vi "Minhee Analysis.vi"(5 "Data type":T4 items=["AXON", "HEKA", "TEXT"], 7 "Path of File":path=path "C:/Users/KimYG/Desktop/test4.abf") -> ()   [LabVIEW 2017]
uses:
  Data type_new.ctl
  <vilib>/Utility/config.llb/Config Data RefNum.ctl
  Polarity.ctl
  <vilib>/Utility/sysdir.llb/System Directory Type.ctl
  Minhee analysis parameter_new.ctl
  <vilib>/Utility/miscctls.llb/LVRowAndColumnTypeDef.ctl
  <vilib>/Analysis/3filter.llb/Savitzky-Golay Filter (DBL).vi
  <vilib>/addons/Wavelet Analysis/application.llb/WA Multiscale Peak Detection (Array).vi
  <vilib>/Utility/file.llb/Write Delimited Spreadsheet (DBL).vi
  <vilib>/Analysis/NI_AALBase.lvlib
  <vilib>/addons/_Advanced Signal Processing/NI_AdvSigProcWA.lvlib
  <vilib>/Utility/config.llb/NI_LVConfig.lvlib
  <vilib>/Analysis/NI_AALPro.lvlib
panel:
  out "History log":string
  in  "Offset":bool
  in  "Event Detection Parameter":cluster{"Minimal Amplitude":dbl, "Polarity":T1} {"Polarity" items=["Inward", "Outward"]}
  in  "Screening Parameters":cluster{"Velocity threshold":dbl, " * SD":dbl}
  in  "Redetect":bool
  in  "Derivative":u16(ring) items=["1st", "2nd"]
  in  "Smoothing Parameters":T2={"Polynomial order"=3, "Side points"=35}
  in  "Trace to display":u16(ring) items=["Raw", "Smoothed"]
  out "Averaged Amplitude":dbl[][](graph)
  out "SD of dv/dt":sgl[](graph)
  in  "File Explorer":bool
  in  "Number of Event":i32
  out "StateFileRefnum":T3
  out "End (sec)":string caption="String"
  out "Event":cluster{dbl[], dbl[]}[](graph)
  out "Holding Current":sgl[](graph)
  out "Frequency":string caption="String"
  out "Sweep duration":dbl
  in  "Clipboard":bool
  out "Number of event":i32[][](graph)
  out "Event #":string caption="String"
  out "Begin (sec)":string caption="String"
  out "IEI (sec)":string caption="String"
  out "Amplitude\n     (pA)":string caption="String"
  out "Event #":string caption="String"
  in  "Pin here":bool
  in  "Raw trace":bool
  out "Distribution of amplitude 2":T5(graph) caption="Selected"
  out "Distribution of IEI 2":T5(graph) caption="Selected"
  out "IEI (sec)":string caption="String"
  out "Amplitude\n     (pA)":string caption="String"
  out "CV":sgl[](graph)
  in  "Screening":bool
  out "Derivative of the event":cluster{"X (time)":dbl[], "dX/dt":dbl[]}[](graph)
  in  "Save":bool
  out "Distribution of amplitude":T5(graph) caption="Total"
  out "Distribution of IEI":T5(graph) caption="Total"
  in  "Event #":i16=4 min=0 max=0 step=1
  in  "Delete":bool
  in  "Import":bool
  in  "Sweep #":i32 min=0 max=49 step=1
  out "Event table":string[][](table)
  out "Whole trace":cluster{"Ramp Pattern":dbl[], "X":dbl[]}[](graph)
  # "Result - Total & Selected events"
  # "OFF"
  # "ON"
  # "Total"
  # "Sweep Info."
  # "Event detection parameters"
  # "Action"
  # "Selected"
  # "Smoothing parameters"
  # "Event Table"
  # "Screening parameters"
  # "Explore your data"
  # "Pg Up"
  # "Event"
  # "Pg Dn"
  # "Home"
  # "Sweep"
  # "End"
  # "Number of event to select"
  # "Whole trace"
  # "(pA)"
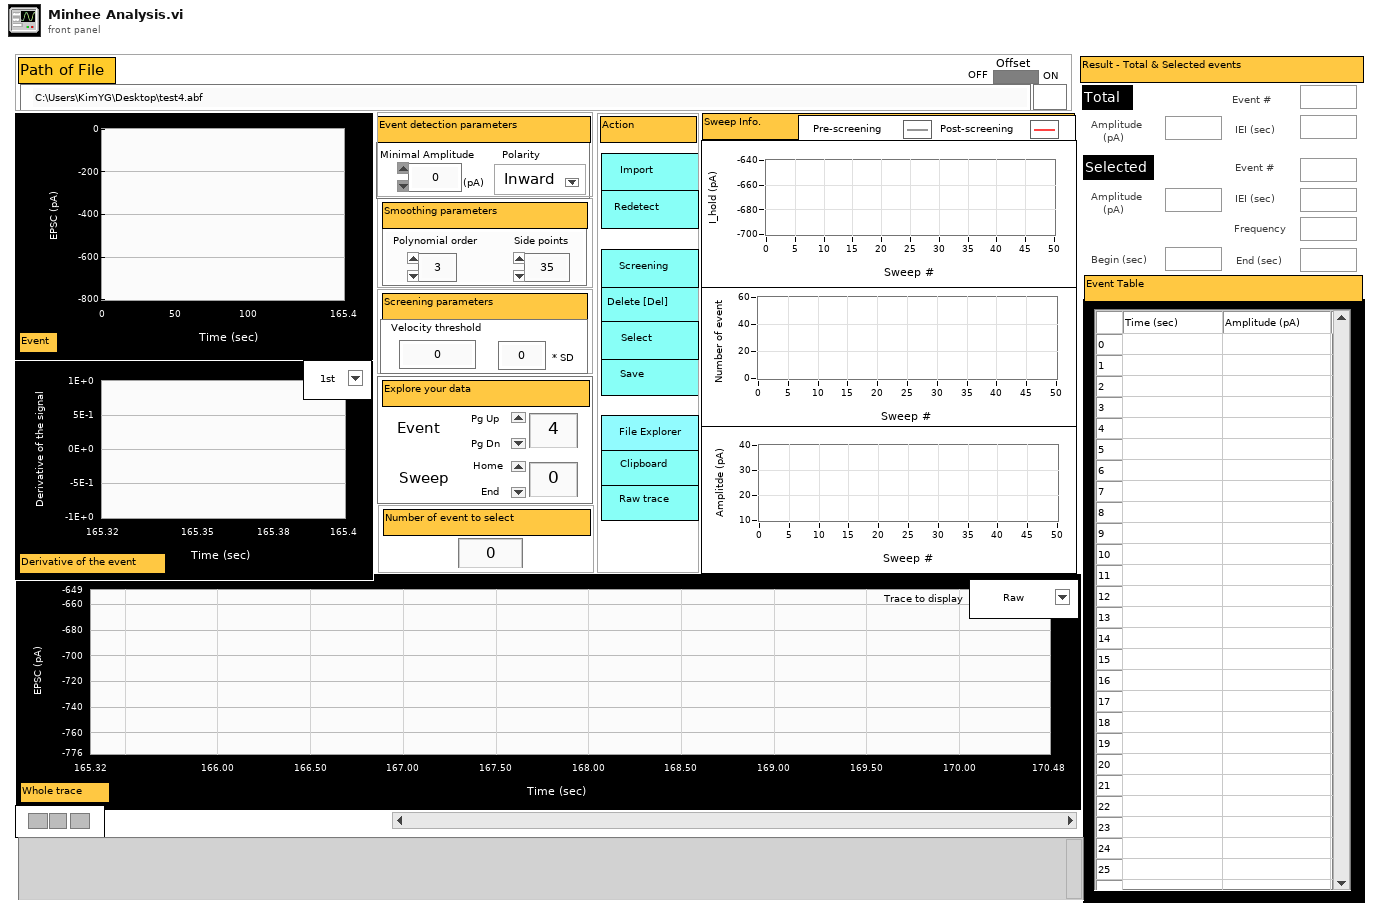
[diagram p1: front panel]
types:
  T1 = typedef "Polarity.ctl" = u16
  T2 = cluster{"Polynomial order":i32, "Side points":i32}
  T3 = typedef "NI_LVConfig.lvlib/Config Data RefNum.ctl" = refnum<k1>
  T4 = typedef "Data type_new.ctl" = u16
  T5 = cluster{"X Values":dbl[], "Histogram: h(x)":i32[]}
  T6 = typedef "Minhee analysis parameter_new.ctl" = cluster{"File Paramters":cluster{"File Path":path, "File Name":string, "Total Length":i32, "Trial Length (ms)":dbl, "Sweep Number":dbl, "Sampling rate":dbl, "Data type":T4}, "Smoothing Parameter":cluster{"Polynomial order":i32, "Side points":i32}, "Event Detection Parameter":cluster{"Event threshold (amplitude)":dbl, "Polarity":T1}, "Screening":cluster{"Screening threshold (dV/dt)":dbl, " * SD":dbl}}
  T7 = cluster{"Total":cluster{"Distribution of IEI":cluster{"X Values":dbl[], "Histogram: h(x)":i32[]}, "Distribution of amplitude":cluster{"X Values":dbl[], "Histogram: h(x)":i32[]}, "Total":cluster{"EVT #":string, "Amplitude":string, "IEI":string}, "Number of event":i32[]}, "Selected":cluster{"Distribution of IEI ":cluster{"X Values":dbl[], "Histogram: h(x)":i32[]}, "Distribution of amplitude":cluster{"X Values":dbl[], "Histogram: h(x)":i32[]}, "Selected":cluster{"EVT #":string, "Amplitude":string, "IEI":string, "Frequency":string}}}
  T8 = cluster{"Distribution of IEI ":cluster{"X Values":dbl[], "Histogram: h(x)":i32[]}, "Distribution of amplitude":cluster{"X Values":dbl[], "Histogram: h(x)":i32[]}, "Selected":cluster{"EVT #":string, "Amplitude":string, "IEI":string, "Frequency":string}}
  T9 = cluster{"detrend? (F)":bool, "threshold frequency":dbl}
  T10 = typedef "System Directory Type.ctl" = i32
  T11 = cluster{"X (time)":dbl[], "I (pA)":dbl[], "dX/dt":dbl[]}
  T12 = typedef "LVRowAndColumnTypeDef.ctl" = cluster{"Row":i32, "Column":i32}
  T13 = cluster{"Sampling rate (Hz)":dbl, "Sweep duration (sec)":dbl, "Unit (A or pA)":u16, "Baseline Offset (pA)":dbl}
  T14 = cluster{"File Path":path, "Cell ID":string, "File Name":string, "Total Length":i32, "Trial Length (ms)":dbl, "Sweep Number":dbl, "Sampling rate":dbl}
  T15 = cluster{"IEI histogram":cluster{"X Values":dbl[], "Histogram: h(x)":i32[]}, "Amplitude histogram":cluster{"X Values":dbl[], "Histogram: h(x)":i32[]}, "Result in Total ":cluster{"Event #":string, "Amplitude ":string, "IEI":string}, i32[]}
  T16 = cluster{"Polynomial order":i32, "Side points":i32}[]
  T17 = cluster{"Histogram Graph":cluster{"X Values":dbl[], "Histogram: h(x)":i32[]}, "Histogram Graph":cluster{"X Values":dbl[], "Histogram: h(x)":i32[]}, cluster{string, "standard deviation":string, "standard deviation":string}, i32[]}
  T18 = cluster{"Histogram Graph":cluster{"X Values":dbl[], "Histogram: h(x)":i32[]}, "Histogram Graph":cluster{"X Values":dbl[], "Histogram: h(x)":i32[]}, cluster{"EVT #":string, "Mean amplitude":string, "Mean IEI":string, "Mean frequency":string}}
  T19 = cluster{"EVT #":string, "Amplitude":string, "IEI":string}
  T20 = cluster{"EVT #":string, "Amplitude":string, "IEI":string, "Frequency":string}
  T21 = cluster{"X (time)":dbl[], "I (pA)":dbl[], "1st derivative":dbl[], "2nd derivative":dbl[]}
  T22 = cluster{"X (time)":dbl[], "2nd derivative":dbl[]}
  T23 = cluster{"X (time)":dbl[], "2nd derivative":dbl[]}[]
  T24 = enum32{"invalid app kind", "Development System", "Run Time System", "Student Edition", "Embedded LabVIEW", "Evaluation", "Custom"}
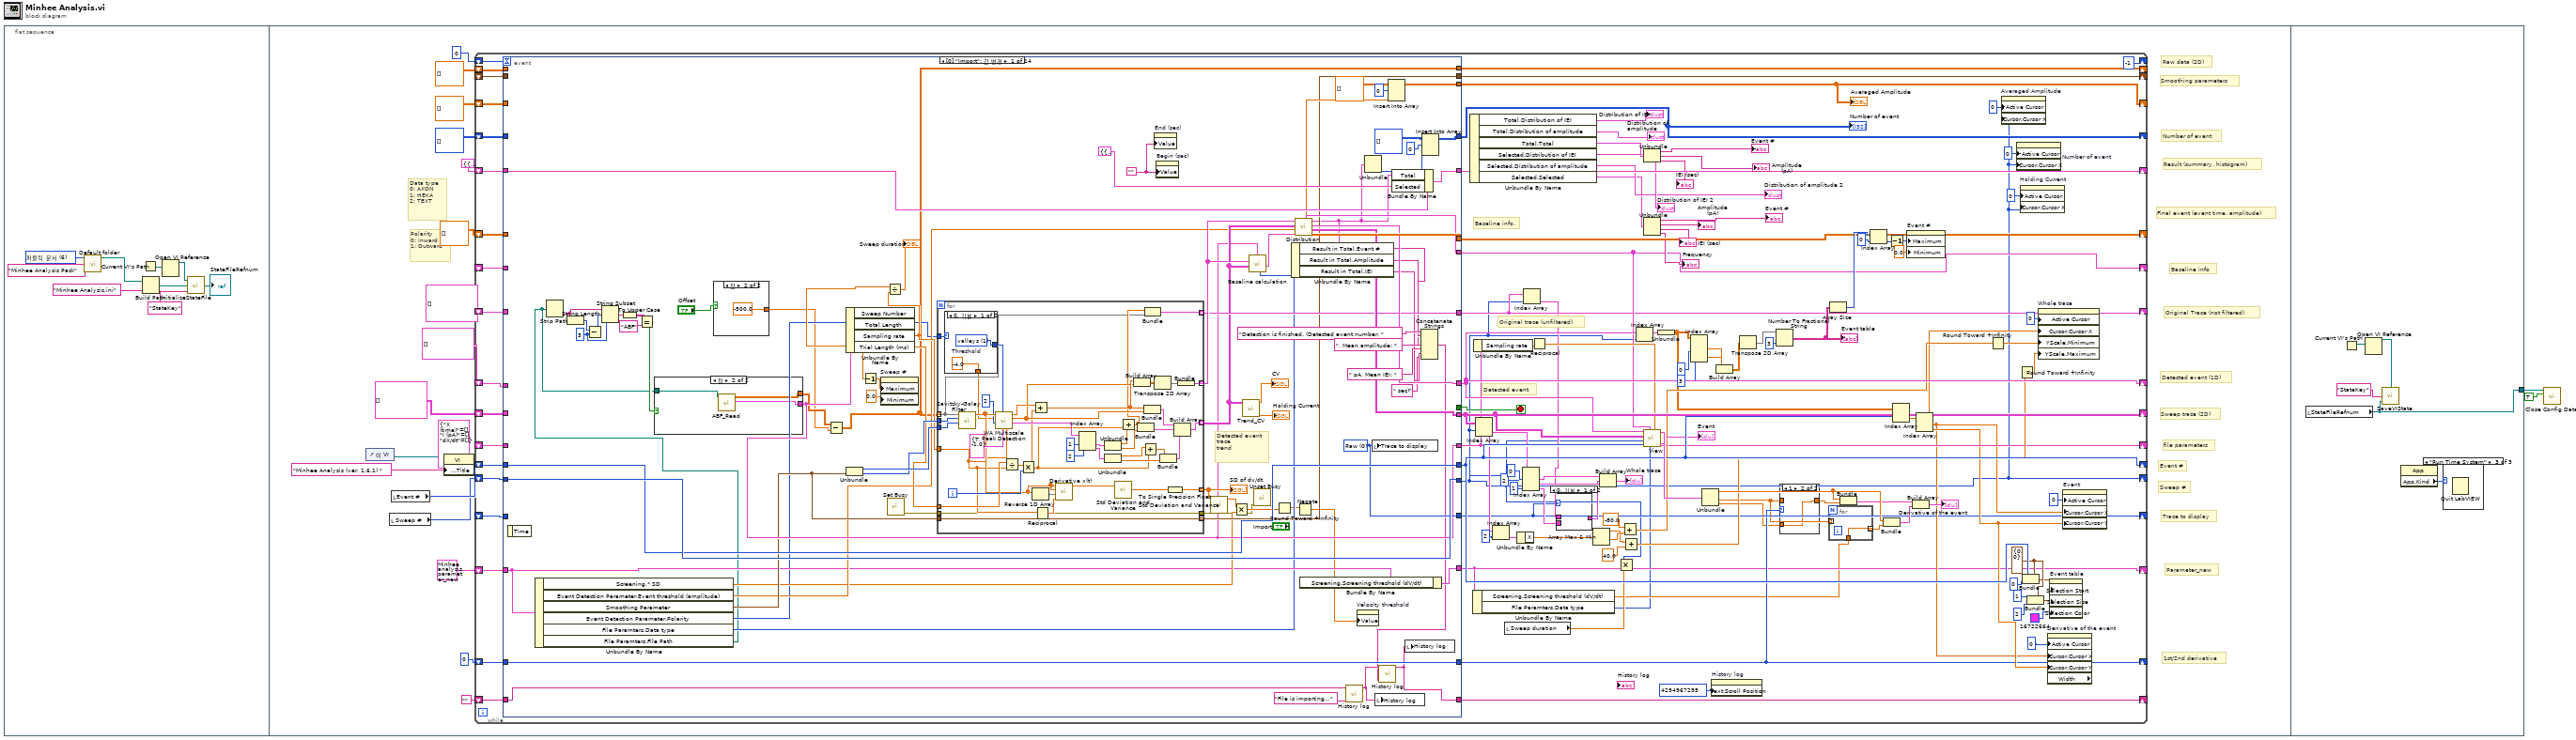
[diagram p0: block diagram]
diagram:
  n1 = flat-sequence {
    tunnel: [w730] -> w1
    frame #0 {
      w9 = T10 6 items=["사용자 홈"=0, "사용자 데스크탑"=1, "사용자 문서"=2, "사용자 어플리케이션 데이터"=3, "사용자 환경"=4, "사용자 임시"=5, "퍼블릭 문서"=6, "퍼블릭 어플리케이션 데이터"=7, "퍼블릭 환경"=8, "퍼블릭 캐시"=13, "시스템 코어 라이브러리"=9, "시스템 설치된 라이브러리"=10, "어플리케이션 파일"=11, "부팅 볼륨 루트"=12] ("system directory type")
      n2 = call <userlib>:"Default folder.vi"("Folder name"="Minhee Analysis Pack", "system directory type"=w9) -> ("Folder path"=w11:path)  [unwired: 5 in]
      n3 = Current VI's Path ("Current VI Path...")() -> (path=w7:path)
      n4 = Build Path(base path=w11, name or relative path="Minhee Analysis.ini") -> (appended path=w3:path)
      n5 = Open VI Reference(vi path=w7) -> (vi reference=w6:refnum<vi>)  [unwired: 5 in, 1 out]
      n6 = call <userlib>:"InitializeStateFile.vi"("key"="StateKey", "configuration file path"=w3, "VI Refnum"=w6) -> ("StateFileRefnum"=→"StateFileRefnum":T3)
    }
    frame #1 {
      (unwired) cluster{dbl[], dbl[]}[] []
      (unwired) T11 {"X (time)"=[], "I (pA)"=[], "dX/dt"=[]} ("출력 클러스터")
      # "Parameter_new"
      # "Final event (event time, amplitude)"
      # "1st/2nd derivative"
      # "Smoothing parameters"
      # "Raw data (2D)"
      # "Trace to display"
      # "Original Trace (not filtered)"
      # "Baseline info"
      # "Polarity \n0: Inward\n1: Outward"
      # "Data type \n0: AXON\n1: HEKA\n2: TEXT"
      # "file parameters"
      # "Number of event"
      # "Result (summary, histogram)"
      # "Sweep trace (2D)"
      # "Detected event (1D)"
      # "Event #"
      # "Sweep #"
      n7 = control-ref of="이 VI"() -> (w15:refnum<vi>)
      n8 = local read "Sweep #"() -> (w16:i32)
      n9 = local read "Event #"() -> (w17:i16)
      n10 = property class="VI"(reference=w15, "Front Panel.Title"="Minhee Analysis (ver. 1.6.1) " ("프런트패널 윈도우:제목")) -> ()  [unwired: 1 in, 2 out]
      n11 = while {
        shift-right: [w137] -> _
        shift-left: cluster{"Ramp Pattern":dbl[], "X":dbl[]}[][] [] ("peak plot") -> [w143]
        shift-right: [w37] -> _
        shift-left: w16 -> [w144]
        shift-right: [w133] -> _
        shift-left: cluster{dbl[][]}[] [] -> [w141]
        shift-right: [w120] -> _
        shift-left: w17 -> [w139]
        shift-right: [w109] -> _
        shift-left: dbl[][] [] ("Event final") -> [w108]
        shift-right: [w103] -> _
        shift-left: T7 {"Total"={"Distribution of IEI"={"X Values"=[], "Histogram: h(x)"=[]}, "Distribution of amplitude"={"X Values"=[], "Histogram: h(x)"=[]}, "Total"={"EVT #"="", "Amplitude"="", "IEI"=""}, "Number of event"=[]}, "Selected"={"Distribution of IEI "={"X Values"=[], "Histogram: h(x)"=[]}, "Distribution of amplitude"={"X Values"=[], "Histogram: h(x)"=[]}, "Selected"={"EVT #"="", "Amplitude"="", "IEI"="", "Frequency"=""}}} -> [w104]
        shift-right: [w89] -> _
        shift-left: i32[][] [] -> [w90]
        shift-right: [w87] -> _
        shift-left: _ -> [w88]
        shift-right: [w76] -> _
        shift-left: _ -> [w77]
        shift-right: [w71] -> _
        shift-left: _ -> [w74]
        shift-right: [w62] -> _
        shift-left: dbl[][] [] ("Event final") -> [w63]
        shift-right: [w56] -> _
        shift-left: _ -> [w57]
        shift-right: [w55] -> _
        shift-left: dbl[][] [] ("Whole Trace") -> [w54]
        shift-right: [w53] -> _
        shift-left: _ -> [w52]
        shift-right: [w50] -> _
        shift-left: u16 0 ("Derivative") -> [w51]
        shift-right: [w34] -> _
        shift-left: T6 {"File Paramters"={"File Path"=path "", "File Name"="", "Total Length"=0, "Trial Length (ms)"=0.0, "Sweep Number"=0.0, "Sampling rate"=0.0, "Data type"=0}, "Smoothing Parameter"={"Polynomial order"=3, "Side points"=20}, "Event Detection Parameter"={"Event threshold (amplitude)"=-10.0, "Polarity"=0}, "Screening"={"Screening threshold (dV/dt)"=0.0, " * SD"=2.5}} ("Parameter setting") -> [w35]
        shift-right: [-1] -> _
        shift-left: 0 -> [w31]
        shift-right: [w29] -> _
        shift-left: "" -> [w28]
        stop <- w142 stop-if-true
        w116 = T12 {"Row"=0, "Column"=0} ("선택 시작")
        # "Detected event"
        # "Baseline info."
        # "Original trace (unfiltered)"
        n12 = event shown="[0] \"Import\": 값 변경" {
          selector: _ -> [_ _ _ _ _ _ _ _ _ _ _ _ _ _]
          dyn-events: _ -> [_ _ _ _ _ _ _ _ _ _ _ _ _ _]
          timeout: w31 -> [_ _ _ _ _ _ _ _ _ _ _ _ _ _]
          tunnel: [w209 w299 w341 w407 w436 w466 w490 w522 w549 w561 w579 w614 w651 w687] -> w137
          tunnel: [w204 w296 w315 w405 w448 "Sweep #" w472 w520 w539 w558 w576 w613 w653 w684] -> w37
          tunnel: w144 -> [w204 w296 w315 w405 w448 _ w472 w520 w539 w558 w576 w613 w653 w693]
          tunnel: w143 -> [_ w299 w342 w407 w446 w466 w499 w522 w549 w561 w579 w614 w651 w688]
          tunnel: [_ _ _ _ _ _ _ _ _ _ _ _ _ w701] -> w142
          tunnel: [w210 w300 w330 w406 w434 w465 w489 w523 w548 w562 w580 w616 w650 w689] -> w133
          tunnel: w141 -> [_ w300 w334 w406 w438 w465 w500 w523 w548 w562 w580 w616 w650 w696]
          tunnel: [w203 w297 w353 w402 w447 w459 w476 w521 "Event #" w559 w577 w617 w652 w685] -> w120
          tunnel: w139 -> [w203 w297 w353 w402 w447 _ w476 w521 _ w559 w577 w617 w652 w694]
          tunnel: [w223 w303 w331 w398 w445 w464 w496 w513 w546 w564 w583 w615 w642 w690] -> w109
          tunnel: w108 -> [_ w303 _ w391 _ w464 _ w513 w546 w564 w583 w615 w642 w697]
          tunnel: w104 -> [w222 w304 w329 w388 w444 w463 w494 w524 w547 w565 w584 w597 w638 w698]
          tunnel: [w221 w304 w328 w386 w443 w463 w493 w524 w547 w565 w584 w597 w638 w691] -> w103
          tunnel: w90 -> [_ w305 w323 w385 w442 w462 w498 w525 w540 w566 w585 w596 w637 w699]
          tunnel: [w220 w305 w324 w385 w441 w462 w498 w525 w540 w566 w585 w596 w637 w692] -> w89
          tunnel: [w180 w298 w321 w384 w425 w461 w484 w515 w545 w560 w578 w595 w636 w686] -> w87
          tunnel: w88 -> [_ w298 w321 w384 w425 w461 w484 w515 w545 w560 w578 w595 w636 w695]
          tunnel: [w205 w302 w332 w382 w432 w460 w488 w512 w544 w556 w582 w594 w635 w681] -> w76
          tunnel: w77 -> [_ w302 w339 w382 _ w460 _ w512 w544 w556 w582 w594 w635 w682]
          tunnel: [w201 w301 w354 w370 w431 w458 w487 w511 w543 w563 w581 w593 w634 w679] -> w71
          tunnel: w74 -> [_ w301 w354 w370 w431 w458 w487 w511 w543 w563 w581 w593 w634 w680]
          tunnel: w63 -> [_ w306 w336 w368 w429 w457 w486 w510 w542 w567 w575 w592 w632 w678]
          tunnel: [w194 w306 w335 w368 w428 w457 w486 w510 w542 w567 w575 w592 w632 w677] -> w62
          tunnel: [w191 w295 w352 w367 w426 w456 w485 w509 w541 "Trace to display" w574 w591 w631 w675] -> w56
          tunnel: w57 -> [_ w295 w352 w367 w426 w456 w485 w509 w541 _ w574 w591 w631 w676]
          tunnel: [w165 w308 w349 w366 w424 w455 w483 w508 w538 w555 w573 w590 w630 w673] -> w55
          tunnel: w54 -> [_ w308 w349 w366 w424 w455 w483 w508 w538 w555 w573 w590 w630 w674]
          tunnel: [w189 w307 w350 w365 w423 w454 w482 w507 w537 w554 w572 w589 w629 w671] -> w53
          tunnel: w52 -> [_ w307 w351 w365 w423 w454 w482 w507 w537 w554 w572 w589 w629 w672]
          tunnel: [w188 w294 w348 w364 w422 w451 w481 w506 w536 "Derivative" w571 w588 w628 w669] -> w50
          tunnel: w51 -> [w188 w294 w348 w364 w422 w451 w481 w506 w536 _ w571 w588 w628 w670]
          tunnel: w35 -> [w175 w293 w319 w363 w420 w450 w480 w505 w535 w552 w570 w587 w627 w666]
          tunnel: [w174 w288 w319 w363 w420 w450 w480 w505 w535 w552 w570 w587 w627 w665] -> w34
          tunnel: [w161 w284 w309 w361 w411 w449 w468 w501 w534 w551 w568 w586 w618 w663] -> w29
          tunnel: w28 -> [w164 w286 w316 w362 w417 w449 w477 w503 w534 w551 w568 w586 w624 w664]
          event "Import": Value Change {
            w184 = 3 ("y")
            w191 = u16 0 items=["Raw", "Smoothed"] ("Trace to display")
            w202 = ""
            # "Detected event\ntrace\ntrend"
            n13 = event-data() -> ()  [unwired: 1 in, 1 out]
            n14 = Unbundle By Name(w175) -> ("Screening.* SD"=w176:dbl, "Event Detection Parameter.Event threshold (amplitude)"=w177:dbl, "Smoothing Parameter"=w178:T2, "Event Detection Parameter.Polarity"=w173:T1, "File Paramters.Data type"=w172:T4, "File Paramters.File Path"=w171:path)
            n15 = Strip Path(path=w171) -> (name=w187:string)  [unwired: 1 out]
            n16 = String Length(string=w187) -> (length=w186:i32)
            n17 = Subtract(x=w186, y=w184) -> (x-y=w185:i32)
            n18 = String Subset(string=w187, offset (0)=w185, length (rest)=w184) -> (substring=w183:string)
            n19 = To Upper Case(1:w183) -> (0:w182:string)
            n20 = Equal?(x=w182, y="ABF") -> (x = y?=w179:bool)
            n21 = case shown="참" w179 {
              tunnel: [w233 w235] -> w168
              tunnel: w171 -> [w232 w236]
              tunnel: [w228 w234] -> w180
              frame False {
                n22 = call "Additional config for txt file.vi"() -> ("Configuration for text file"=w231:T13)  [unwired: 4 in]
                n23 = Unbundle By Name(w231) -> ("Sampling rate (Hz)"=w230:dbl)
                n24 = call "TXT_Read.vi"("Configuration for text file"=w231, "Path of ABF file"=w232) -> ("File Paramters"=w229:T14, "Whole Trace"=w233:sgl[][])  [unwired: 2 in, 2 out]
                n25 = Bundle By Name(cluster=w229, "Sampling rate"=w230) -> (w228:T14)
              }
              frame True {
                n26 = call "ABF_Read.vi"("Path of ABF file"=w236) -> ("File Paramters"=w234:T14, "Whole Trace"=w235:sgl[][])  [unwired: 4 in, 1 out]
              }
            }
            n27 = case shown="참" "Offset" {
              tunnel: [0.0 ("데이터 입력 제한:최소") -500.0 ("데이터 입력 제한:최소")] -> w166
              frame False {
              }
              frame True {
              }
            }
            n28 = Subtract(x=w168, y=w166) -> (x-y=w165:dbl[][])
            n29 = Unbundle By Name(w180) -> ("Sweep Number"=w216:dbl, "Sampling rate"=w200:dbl, "Trial Length (ms)"=w214:dbl)  [unwired: 1 out]
            n30 = Unbundle(w178) -> ("Polynomial order"=w225:i32, "Side points"=w224:i32)
            n31 = Decrement(x=w216) -> (x-1=w217:dbl)
            n32 = property on="Sweep #" class="DigNum (엄격한)"("Maximum"=w217, "Minimum"=0.0 ("데이터 입력 제한:최소")) -> ()  [unwired: 2 in, 2 out]
            n33 = Divide(x=w214, y=w200) -> (x/y=→"Sweep duration":dbl)
            n34 = call <vilib>:"Set Busy.vi"() -> ("error out"=w151:errorcluster)  [unwired: 10 in, 1 out]
            n35 = for {
              tunnel: w165 -> [w249] mode=indexing
              tunnel: w200 -> [w245]
              tunnel: w224 -> [w277]
              tunnel: w225 -> [w276]
              tunnel: [w254] -> w190 mode=indexing
              tunnel: w214 -> [w268]
              tunnel: [w271] -> w206 mode=indexing
              tunnel: w173 -> [w251]
              tunnel: [w248] -> w201 mode=indexing
              tunnel: [w240] -> w199 mode=indexing
              tunnel: w178 -> [w242]
              tunnel: [w242] -> w189 mode=indexing
              tunnel: w151 -> [w237]
              tunnel: [w237] -> w150
              i -> [w252]
              n36 = case shown="0, 기본" w251 {
                tunnel: [w281 w283] -> w279
                tunnel: [w280 w282] -> w238
                frame 0, Default {
                  w280 = -4.0  # Threshold
                  w281 = u16 1 items=["peaks", "valleys"] ("peaks/valleys")
                }
                frame 1 {
                  w282 = 4.0  # Threshold
                  w283 = u16 0 items=["peaks", "valleys"] ("peaks/valleys")
                }
              }
              n37 = call-poly <vilib>:"Savitzky-Golay Filter.vi"("polynomial order"=w276, "side points"=w277, "X"=w249) -> ("Filtered X"=w247:dbl[])  [unwired: 7 in, 1 out]
              n38 = call-poly <vilib>:"WA Multiscale Peak Detection.vi"("sampling rate"=w245, "detrend settings"=T9 {"detrend? (F)"=TRUE, "threshold frequency"=-1.0}, "peaks/valleys"=w279, "width"=2 ("인덱스"), "threshold"=w238, "signal"=w247) -> ("peak plot"=w267:cluster{"Ramp Pattern":dbl[], "X":dbl[]}[], "amplitude"=w269:dbl[], "location"=w274:dbl[])  [unwired: 1 in, 2 out]
              n39 = Divide(x=w268, y=w245) -> (x/y=w275:dbl)
              n40 = Multiply(x=w275, y=w252) -> (x*y=w253:dbl)
              n41 = Reverse 1D Array(array=w247) -> (reversed array=w246:dbl[])
              n42 = Add(x=w274, y=w253) -> (x+y=w270:dbl[])
              n43 = Reciprocal(x=w245) -> (1/x=w244:dbl)
              n44 = call <vilib>:"Derivative x(t).vi"("dt"=w244, "Final Condition"=w246, "Initial Condition"=w247, "X"=w247) -> ("dX/dt"=w243:dbl[])  [unwired: 6 in, 1 out]
              n45 = Index Array(array=w267, index #1=1 ("인덱스"), index #2=2 ("인덱스")) -> (element #1=w265:cluster{"Ramp Pattern":dbl[], "X":dbl[]}, element #2=w261:cluster{"Ramp Pattern":dbl[], "X":dbl[]})
              n46 = Unbundle(w265) -> ("Ramp Pattern"=w264:dbl[], "X"=w263:dbl[])
              n47 = Unbundle(w261) -> ("Ramp Pattern"=w260:dbl[], "X"=w258:dbl[])
              n48 = call <vilib>:"Std Deviation and Variance.vi"("X"=w243) -> ("standard deviation"=w241:dbl)  [unwired: 1 in, 2 out]
              n49 = Add(x=w264, y=w253) -> (x+y=w250:dbl[])
              n50 = Build Array(w270, w269) -> (w273:dbl[][])
              n51 = Bundle(w250, "X"=w263) -> (w256:cluster{dbl[], "X":dbl[]})  [unwired: 1 in]
              n52 = Add(x=w260, y=w253) -> (x+y=w259:dbl[])
              n53 = Bundle(w270, "amplitude"=w269) -> (w255:cluster{dbl[], "amplitude":dbl[]})  [unwired: 1 in]
              n54 = Bundle(w250, w249) -> (w248:cluster{dbl[], dbl[]})  [unwired: 1 in]
              n55 = Transpose 2D Array(2D array=w273) -> (transposed array=w272:dbl[][])
              n56 = Bundle(w259, "X"=w258) -> (w257:cluster{dbl[], "X":dbl[]})  [unwired: 1 in]
              n57 = To Single Precision Float(number=w241) -> (single precision float=w240:sgl)
              n58 = Build Array(w255, w256, w257) -> (w254:cluster{dbl[], "X":dbl[]}[])
              n59 = Bundle(w272) -> (w271:cluster{dbl[][]})  [unwired: 1 in]
            }
            "SD of dv/dt" <- w199
            n60 = property on="End (sec)" class="Str"("Value"=w202) -> ()  [unwired: 2 in, 2 out]
            n61 = property on="Begin (sec)" class="Str"("Value"=w202) -> ()  [unwired: 2 in, 2 out]
            n62 = call <vilib>:"Std Deviation and Variance.vi"("X"=w199) -> ("mean"=w198:dbl)  [unwired: 1 in, 2 out]
            n63 = Multiply(x=w198, y=w176) -> (x*y=w197:dbl)
            n64 = call "Trend_CV.vi"("Original trace (1D)"=w190) -> ("Holding Current (pA)"=→"Holding Current":sgl[], "CV"=→"CV":sgl[])  [unwired: 5 in]
            n65 = call "Baseline calculation.vi"("Data type"=w172, "File Paramters"=w180, "Sweep trace (2D) In"=w190, "Detected Event (1D) In"=w206) -> ("New Baseline info"=w192:cluster{dbl[][]}[])  [unwired: 6 in, 1 out]
            n66 = call <vilib>:"Unset Busy.vi"("error in (no error)"=w150) -> ()  [unwired: 10 in, 1 out]
            n67 = Round Toward +Infinity(x=w197) -> (ceil(x): smallest int >= x=w170:dbl)
            n68 = call "Distribution.vi"("Detected Event IN"=w206, "Sweep trace (2D) In"=w190, "Threshold"=w177, "Baseline info IN"=w192) -> ("Baseline info new OUT"=w205:cluster{dbl[][]}[], "Averaged amplitude (pA)"=w195:dbl[], "Distribution (output)"=w160:T15, "Detected Event (1D) OUT"=w210:cluster{dbl[][]}[], "Sweep trace (2D) Out"=w209:cluster{"Ramp Pattern":dbl[], "X":dbl[]}[][], "Event final OUT"=w223:dbl[][])
            n69 = Unbundle By Name(w160) -> ("Result in Total.Event #"=w158:string, "Result in Total.Amplitude"=w156:string, "Result in Total.IEI"=w154:string)
            n70 = Negate(x=w170) -> (-x=w169:dbl)
            n71 = Bundle By Name(cluster=w175, "Screening.Screening threshold (dV/dt)"=w169) -> (w174:T6)
            n72 = call "History log.vi"("Message"="File is importing...", "String IN"=w164) -> ("String OUT"=w162:string)  [unwired: 5 in]
            n73 = property on="Velocity threshold" class="DigNum (엄격한)"("Value"=w169) -> ()  [unwired: 2 in, 2 out]
            n74 = Unbundle(w160) -> (w218:i32[])  [unwired: 3 out]
            n75 = local write "Trace to display"(w191) -> ()
            n76 = local write "History log"(w162) -> ()
            n77 = Insert Into Array(array=sgl[][] [] ("Event final"), index (row)=0 ("인덱스 (행)"), new element=w195) -> (w194:sgl[][])  [unwired: 1 in]
            n78 = Bundle By Name(cluster=w222, "Total"=w160, "Selected"=T8 {"Distribution of IEI "={"X Values"=[], "Histogram: h(x)"=[]}, "Distribution of amplitude"={"X Values"=[], "Histogram: h(x)"=[]}, "Selected"={"EVT #"="", "Amplitude"="", "IEI"="", "Frequency"=""}}) -> (w221:T7)
            n79 = Concatenate Strings("Detection is finished. (Detected event number: " ("문자열"), w158, ", Mean amplitude: " ("문자열"), w156, " pA, Mean IEI: " ("문자열"), w154, " sec)" ("문자열")) -> (w153:string)
            n80 = call "History log.vi"("Message"=w153, "String IN"=w162) -> ("String OUT"=w161:string)  [unwired: 5 in]
            n81 = local write "History log"(w161) -> ()
            n82 = Insert Into Array(array=i32[][] [], index (row)=0, new element=w218) -> (w220:i32[][])  [unwired: 1 in]
          }
          event "Smoothing Parameters", "Path of File", "Screening Parameters", "Event Detection Parameter": Value Change; Timeout {
            n83 = event-data() -> ()  [unwired: 1 in, 1 out]
            n84 = Bundle By Name(cluster=w293, "File Paramters.File Path"="Path of File", "Smoothing Parameter"="Smoothing Parameters", "Screening"="Screening Parameters", "Event Detection Parameter"="Event Detection Parameter", "File Paramters.Data type"="Data type") -> (w288:T6)
            n85 = call "History log.vi"("Message"="Path of File or Event detection/Smoothing/Screening parameters have been changed.", "String IN"=w286) -> ("String OUT"=w284:string)  [unwired: 5 in]
            n86 = local write "History log"(w284) -> ()
          }
          event "Redetect": Value Change {
            n87 = event-data() -> ()  [unwired: 1 in, 1 out]
            n88 = Unbundle By Name(w319) -> ("Smoothing Parameter"=w320:T2, "Event Detection Parameter.Event threshold (amplitude)"=w318:dbl, "File Paramters.Data type"=w317:T4)
            n89 = Index Array(array=w349, index (row)=w315) -> (element=w347:dbl[])  [unwired: 1 in]
            n90 = Replace Array Subset(array=w351, new element=w320, index=w315) -> (w350:T16)
            n91 = call "Redetection_initial detectoin.vi"("Sweep #"=w315, "File Paramters"=w321, "New Smoothing Parameter"=w320, "Data (1 sweep)"=w347, "Polarity"=w317) -> ("Sweep trace"=w345:cluster{dbl[], "X":dbl[]}[], "Detected event"=w344:cluster{dbl[][]})  [unwired: 4 in, 1 out]
            n92 = call "Redetection_Baseline calculation.vi"("Sweep #"=w315, "File Paramters"=w321, "Sweep trace (1D)"=w345, "Detected event"=w344, "Data type"=w317) -> ("New baseline info"=w346:cluster{dbl[][]})  [unwired: 6 in]
            n93 = call "Redetection_Distribution.vi"("Detected Event (1D) IN"=w334, "Sweep trace (1D) IN"=w345, "Threshold"=w318, "Detected event IN"=w344, "New baseline info IN"=w346) -> ("EVT # (redetected)"=w322:i32, "Sweep trace (1D) Out"=w343:cluster{"Ramp Pattern":dbl[], "X":dbl[]}[], "Averaged amplitude (pA)"=w337:dbl, "New baseline info OUT"=w340:cluster{dbl[][]}, "Detected Event OUT"=w333:cluster{dbl[][]})
            n94 = Number To Decimal String(number=w315, width (-)=i16 1 ("폭(-)")) -> (decimal integer string=w313:string)
            n95 = Replace Array Subset(array=w334, new element=w333, index=w315) -> (w330:cluster{dbl[][]}[])
            n96 = Replace Array Subset(array=w342, new element=w343, index (row)=w315) -> (w341:cluster{"Ramp Pattern":dbl[], "X":dbl[]}[][])  [unwired: 1 in]
            n97 = Concatenate Strings("Events are redetected in sweep #", w313, "." ("문자열")) -> (w310:string)
            n98 = Replace Array Subset(array=w336, new element=w337, index (row)=0 ("인덱스 (행)"), index (col)=w315) -> (w335:dbl[][])
            n99 = Replace Array Subset(array=w339, new element=w340, index=w315) -> (w332:cluster{dbl[][]}[])
            n100 = call "History log.vi"("Message"=w310, "String IN"=w316) -> ("String OUT"=w309:string)  [unwired: 5 in]
            n101 = call "Redetection_Final EVT OUT.vi"("Sweep # IN"=w315, "Detected event (1D)"=w330, "EVT # (redetected)"=w322, "Number of event IN"=w323) -> ("Final EVT OUT"=w331:dbl[][], "Distribution (output)"=w327:T17)  [unwired: 2 in]
            n102 = local write "History log"(w309) -> ()
            n103 = Unbundle(w327) -> (w326:i32[])  [unwired: 3 out]
            n104 = Bundle By Name(cluster=w329, "Total"=w327) -> (w328:T7)
            n105 = Replace Array Subset(array=w323, new element=w326, index (row)=0 ("인덱스 (행)")) -> (w324:i32[][])  [unwired: 1 in]
          }
          event "Pin here": Value Change {
            n106 = event-data() -> ()  [unwired: 1 in, 2 out]
            n107 = Index Array(array=w391, index (col) #1=0 ("비활성화된 인덱스 (열)"), index (col) #2=2 ("인덱스 (열)")) -> (element #1=w399:dbl[], element #2=w374:dbl[])  [unwired: 2 in]
            n108 = Array Size(array=w374) -> (size(s)=w372:i32)
            n109 = Greater Or Equal?(x=w372, y="Number of Event") -> (x >= y?=w373:bool)
            n110 = case shown="거짓" w373 {
              tunnel: [w408 w409] -> w371
              tunnel: w372 -> [w408 _]
              tunnel: "Number of Event" -> [_ w409]
              frame False {
              }
              frame True {
              }
            }
            n111 = Index Array(array=w406, index=w405) -> (element=w404:cluster{dbl[][]})
            n112 = Unbundle(w404) -> (w403:dbl[][])
            n113 = Initialize Array(0.0 ("원소"), w372) -> (w392:dbl[])
            n114 = for {
              N: w371 -> [_]
              tunnel: [1.0 ("x")] -> w396 mode=indexing
            }
            n115 = Index Array(array=w403, index (row)=w402) -> (element=w401:dbl[])  [unwired: 1 in]
            n116 = Index Array(array=w401) -> (element=w389:dbl)  [unwired: 1 in]
            n117 = Search 1D Array(1D array=w399, element=w389) -> (index of element=w390:i32)  [unwired: 1 in]
            n118 = Number To Fractional String(number=w389, precision (6)=i16 3 ("정밀도(6)")) -> (F-format string=w359:string)  [unwired: 2 in]
            "Begin (sec)" <- w359
            n119 = Delete From Array(array=w391, length=w371, index (row)=w390) -> (deleted portion=w381:dbl[][])  [unwired: 1 in, 1 out]
            n120 = Index Array(array=w381, index (col)=0 ("비활성화된 인덱스 (열)")) -> (element=w379:dbl[])  [unwired: 1 in]
            n121 = Array Size(array=w379) -> (size(s)=w378:i32)
            n122 = Decrement(x=w378) -> (x-1=w377:i32)
            n123 = Index Array(array=w379, index=w377) -> (element=w375:dbl)
            n124 = call "Section selection.vi"("Length"=w371, "Event final"=w381) -> ("Distribution (output)"=w387:T18)  [unwired: 5 in]
            n125 = Number To Fractional String(number=w375, precision (6)=i16 3 ("정밀도(6)")) -> (F-format string=w357:string)  [unwired: 2 in]
            "End (sec)" <- w357
            n126 = Concatenate Strings("Events between ", w359, "(sec) and " ("문자열"), w357, "(sec) are selected." ("문자열")) -> (w355:string)
            n127 = Replace Array Subset(array=w392, new element=w396, index=w390) -> (w394:dbl[])
            n128 = call "History log.vi"("Message"=w355, "String IN"=w362) -> ("String OUT"=w361:string)  [unwired: 5 in]
            n129 = Bundle By Name(cluster=w388, "Selected"=w387) -> (w386:T7)
            n130 = local write "History log"(w361) -> ()
            n131 = Replace Array Subset(array=w391, new element=w394, index (col)=2 ("비활성화된 인덱스 (열)")) -> (w398:dbl[][])  [unwired: 1 in]
          }
          event "Screening": Value Change {
            w430 = 1
            n132 = event-data() -> ()  [unwired: 1 in, 2 out]
            n133 = Unbundle By Name(w420) -> ("Event Detection Parameter.Event threshold (amplitude)"=w419:dbl, "Screening.Screening threshold (dV/dt)"=w416:dbl, "File Paramters.Data type"=w418:T4)
            n134 = Unbundle By Name(w425) -> ("Sampling rate"=w421:dbl)
            n135 = call "Screening.vi"("Data type"=w418, "Screen threshold (dV/dt)"=w416, "Sampling rate"=w421, "Detected Event (1D) In"=w438, "Sweep trace (2D) In"=w446) -> ("Detected Event (1D) Out"=w435:cluster{dbl[][]}[], "Sweep trace (2D) Out"=w437:cluster{"Ramp Pattern":dbl[], "X":dbl[]}[][])  [unwired: 2 in]
            n136 = call "Baseline calculation.vi"("Data type"=w418, "File Paramters"=w425, "Sweep trace (2D) In"=w437, "Detected Event (1D) In"=w435) -> ("New Baseline info"=w433:cluster{dbl[][]}[])  [unwired: 6 in, 1 out]
            n137 = Number To Decimal String(number=w416) -> (decimal integer string=w414:string)  [unwired: 1 in]
            n138 = call "Distribution.vi"("Detected Event IN"=w435, "Sweep trace (2D) In"=w437, "Threshold"=w419, "Baseline info IN"=w433) -> ("Baseline info new OUT"=w432:cluster{dbl[][]}[], "Averaged amplitude (pA)"=w427:dbl[], "Distribution (output)"=w440:T15, "Detected Event (1D) OUT"=w434:cluster{dbl[][]}[], "Sweep trace (2D) Out"=w436:cluster{"Ramp Pattern":dbl[], "X":dbl[]}[][], "Event final OUT"=w445:dbl[][])
            n139 = Concatenate Strings("Events are filtered by the velocity threshold " ("Message"), w414, "." ("문자열")) -> (w412:string)
            n140 = Unbundle(w440) -> (w439:i32[])  [unwired: 3 out]
            n141 = call "History log.vi"("Message"=w412, "String IN"=w417) -> ("String OUT"=w411:string)  [unwired: 5 in]
            n142 = Bundle By Name(cluster=w444, "Total"=w440) -> (w443:T7)
            n143 = local write "History log"(w411) -> ()
            n144 = Insert Into Array(array=w429, index (row)=w430, new element=w427) -> (w428:dbl[][])  [unwired: 1 in]
            n145 = Insert Into Array(array=w442, index (row)=w430, new element=w439) -> (w441:i32[][])  [unwired: 1 in]
          }
          event "Sweep #": Value Change {
            w459 = i16 0 ("Event #")
            n146 = event-data() -> ()  [unwired: 1 in, 2 out]
            n147 = property on="Event #" class="DigNum (엄격한)"("Value"=w459) -> ()  [unwired: 2 in, 2 out]
            n148 = Index Array(array=w454, index="Sweep #") -> (element=w452:T2)
            n149 = local write "Smoothing Parameters"(w452) -> ()
          }
          event "Delete": Value Change {
            n150 = event-data() -> ()  [unwired: 1 in, 1 out]
            n151 = Unbundle By Name(w480) -> ("Event Detection Parameter.Event threshold (amplitude)"=w479:dbl, "File Paramters.Data type"=w478:T4)
            n152 = call "Delete.vi"("Event #"=w476, "Sweep #"=w472, "Sweep trace (2D) In"=w499, "Detected Event (1D) In"=w500) -> ("Sweep trace (2D) Out"=w491:cluster{"Ramp Pattern":dbl[], "X":dbl[]}[][], "Detected Event (1D) Out"=w497:cluster{dbl[][]}[])  [unwired: 2 in]
            n153 = call "Baseline calculation.vi"("Data type"=w478, "File Paramters"=w484, "Sweep trace (2D) In"=w491, "Detected Event (1D) In"=w497) -> ("New Baseline info"=w492:cluster{dbl[][]}[])  [unwired: 6 in, 1 out]
            n154 = Number To Decimal String(number=w472) -> (decimal integer string=w471:string)  [unwired: 1 in]